vi "Multi-Record Acquisition (Fetch All records)_4xI16_7965R.vi"() -> ()   [LabVIEW 2012]
uses:
  <vilib>/userdefined/High Color/nirio_resource_hc.ctl
  <vilib>/FPGAPlugInAG/PXIe-7965R/niLvFpga_Open_PXIe-7965R.vi
  <vilib>/rvi/interface/common/dynamic/niFpgaDynamicAddResources.vi
  <vilib>/FPGAPlugInAG/Dynamic/niLvFpga_Download_Dynamic.vi
  <vilib>/FPGAPlugInAG/Dynamic/niLvFpga_Run_Dynamic.vi
  <vilib>/Utility/error.llb/Error Cluster From Error Code.vi
  <vilib>/rvi/errors/niLvFpgaAdjustHostInterfaceError.vi
  <vilib>/FPGAPlugInAG/Dynamic/niLvFpga_Close_Dynamic.vi
  <vilib>/rvi/interface/nirviOpenFPGA/nirviOpenFPGA.xnode
  <userlib>/Fast OCT/Debug/Version 1/FPGA Bitfiles/Current/Acquire 2 channel data with DRAM (Multi-Record)_latest.lvbitx
  <vilib>/rvi/interface/nirviMethod/nirviMethod.xnode
  <vilib>/rvi/interface/nirviReadWriteControl/nirviReadWriteControl.xnode
  <vilib>/rvi/interface/nirviCloseFPGA/nirviCloseFPGA.xnode
  <userlib>/FlexRIO Host Library/FlexRIO Host Library (User).lvlib
  <vilib>/rvi/interface/Simulation/niFpgaSimulationCallBeginRW.vi
  NiFpgaLv.dll
panel:
  out "Host FIFO Timed Out?":bool
  out "Buffer Timed Out?":bool
  out "Records Done":u32=500
  out "Elements Remaining":u32
  out "Iterations":i32=4
  in  "Display Raw Data?":bool=TRUE
  out "Channel Data":dbl[][](graph)
  out "Processing Time":u32=2246 format="%.0f ms"
  out "B-Scan Data":dbl[][](graph)
  in  "Device Name":T1="RIO0"
  in  "Stop":bool
  in  "Trigger Type":T2(ring)=enum."External Digital Trigger"
  in  "Record Count":u32=500
  in  "Pre Trigx4":u32=2
  in  "Post  x4":u32=1625
  out "error out":errorcluster
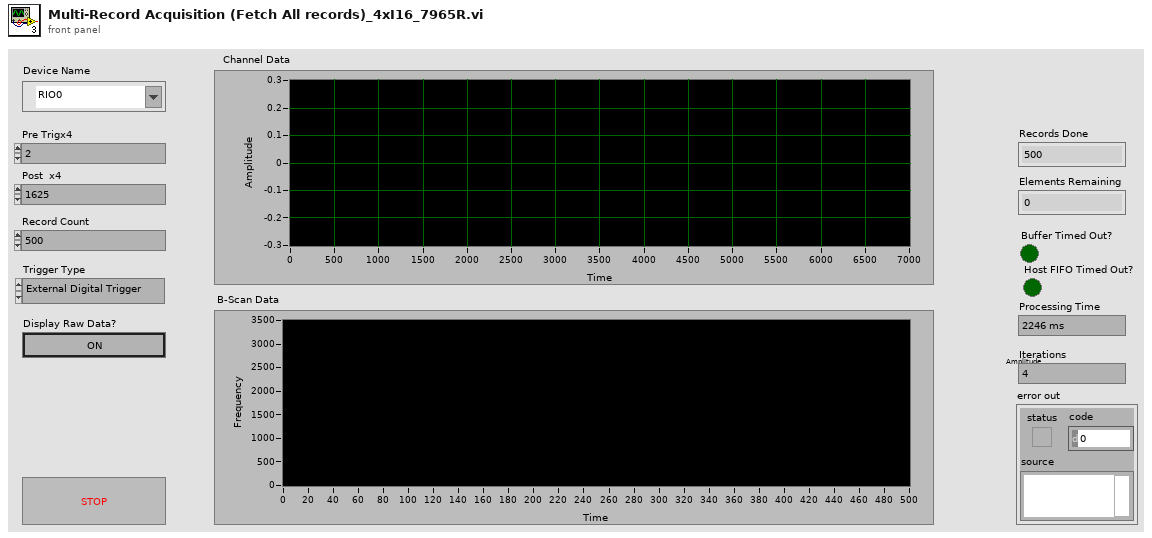
[diagram p1: front panel]
types:
  T1 = typedef "nirio_resource_hc.ctl" = tag
  T2 = enum8{"Immediate Trigger", "Software Trigger", "External Digital Trigger", "Analog Trigger"}
  T3 = cluster{"Load Record Parameters?":bool, "Pre Trigger Samples":u32, "Post Trigger Samples":u32, "Trigger Hold Off":u32, "Record Count":u32}
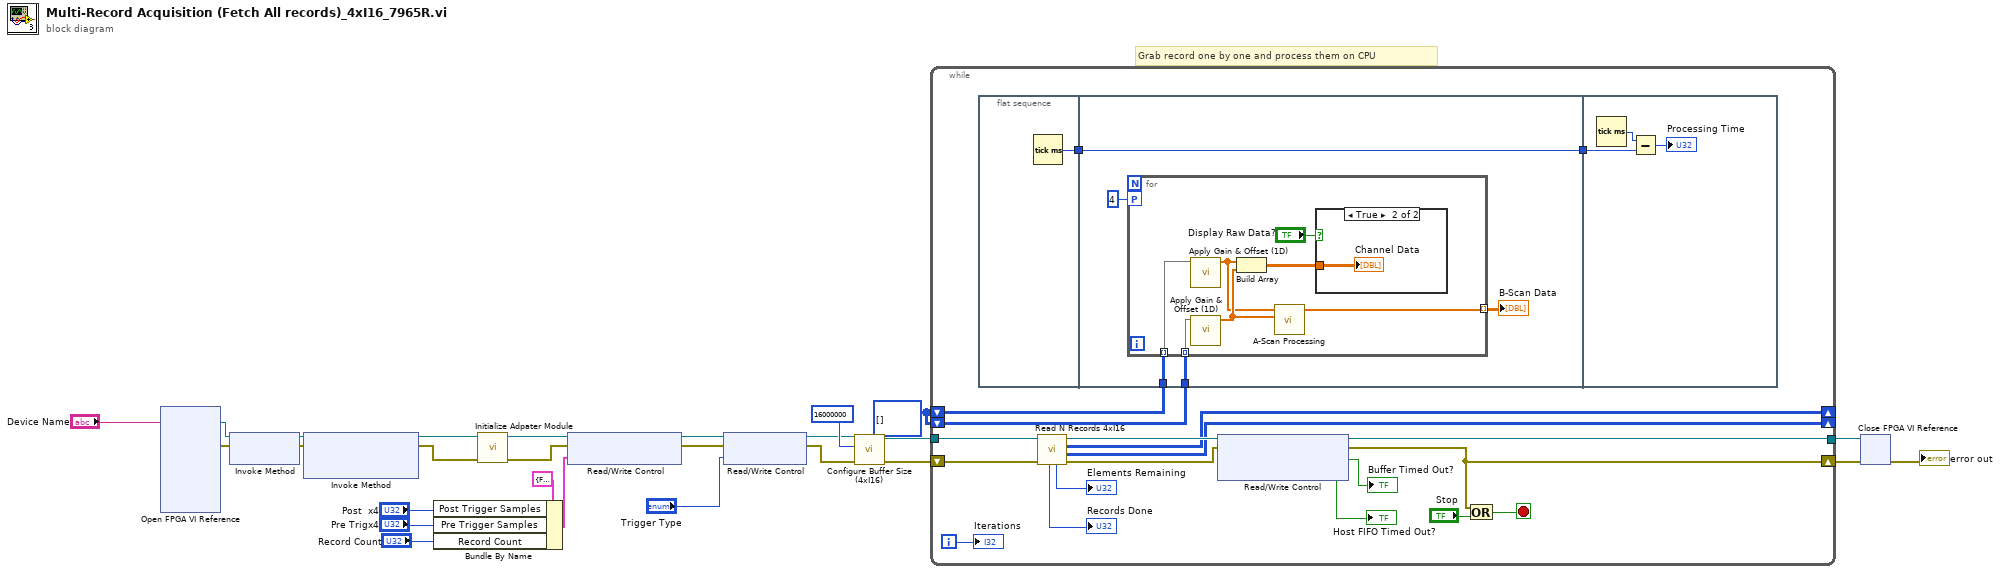
[diagram p0: block diagram]
diagram:
  w1 = i16[][] [] ("Channel 0 Records")
  # "Grab record one by one and process them on CPU"
  n1 = xnode "Open FPGA VI Reference"("resource name"="Device Name") -> ("FPGA VI Reference Out"=w8:refnum<k20>, "error out"=w9:errorcluster)  [unwired: 1 in]
  n2 = xnode "Invoke Method"("FPGA VI Reference In"=w8, "error in"=w9) -> ("FPGA VI Reference Out"=w11:refnum<k20>, "error out"=w10:errorcluster)
  n3 = xnode "Invoke Method"("FPGA VI Reference In"=w11, "error in"=w10) -> ("FPGA VI Reference Out"=w22:refnum<k20>, "error out"=w21:errorcluster)  [unwired: 1 in]
  n4 = Bundle By Name(cluster=T3 {"Load Record Parameters?"=FALSE, "Pre Trigger Samples"=0, "Post Trigger Samples"=0, "Trigger Hold Off"=0, "Record Count"=0} ("Record Parameters"), "Post Trigger Samples"="Post  x4", "Pre Trigger Samples"="Pre Trigx4", "Record Count"="Record Count") -> (w6:T3)
  n5 = call <userlib>:"Initialize Adpater Module.vi"("error in"=w21, "FPGA VI Reference In"=w22) -> ("error out"=w24:errorcluster, "FPGA VI Reference Out"=w25:refnum<k20>)  [unwired: 7 in, 1 out]
  n6 = xnode "Read/Write Control"("FPGA VI Reference In"=w25, "error in"=w24, "Record Parameters"=w6) -> ("FPGA VI Reference Out"=w19:refnum<k20>, "error out"=w18:errorcluster)
  n7 = xnode "Read/Write Control"("FPGA VI Reference In"=w19, "error in"=w18, "Trigger Type"="Trigger Type") -> ("FPGA VI Reference Out"=w14:refnum<k20>, "error out"=w15:errorcluster)
  n8 = call <userlib>:"Configure Buffer Size (4xI16).vi"("error in"=w15, "Buffer Size"=u32 16000000, "FPGA VI Reference In"=w14) -> ("error out"=w4:errorcluster, "FPGA VI Reference Out"=w5:refnum<k20>)  [unwired: 7 in]
  n9 = while {
    tunnel: w5 -> [w45]
    tunnel: [w33] -> w2
    shift-right: [w34] -> w3
    shift-left: w4 -> [w44]
    shift-right: [w30] -> _
    shift-left: w1 -> [w27]
    shift-right: [w29] -> _
    shift-left: w1 -> [w28]
    i -> [w39]
    stop <- w42 stop-if-true
    n10 = flat-sequence {
      tunnel: [w46] -> w41
      tunnel: w41 -> [w50]
      tunnel: [w50] -> w40
      tunnel: w28 -> [w49]
      tunnel: w27 -> [w48]
      tunnel: w40 -> [w61]
      frame #0 {
        n11 = Tick Count (ms)() -> (millisecond timer value=w46:u32)
      }
      frame #1 {
        n12 = for {
          tunnel: [w58] -> w51 mode=indexing
          tunnel: w49 -> [w53] mode=indexing
          tunnel: w48 -> [w52] mode=indexing
          workers-P: 4 -> [_]
          n13 = call <userlib>:"Apply Gain & Offset (1D).vi"("Raw Data"=w53) -> ("Scaled Data"=w55:dbl[])  [unwired: 10 in]
          n14 = call <userlib>:"Apply Gain & Offset (1D).vi"("Raw Data"=w52) -> ("Scaled Data"=w57:dbl[])  [unwired: 10 in]
          n15 = Build Array(w55, w57) -> (w56:dbl[][])
          n16 = call <userlib>:"A-Scan Processing.vi"("K-Clock"=w57, "OCT Signal"=w55) -> ("A-Scan"=w58:dbl[])  [unwired: 9 in]
          n17 = case shown="True" "Display Raw Data?" {
            tunnel: w56 -> [_ w59]
            frame False {
            }
            frame True {
              "Channel Data" <- w59
            }
          }
        }
        "B-Scan Data" <- w51
      }
      frame #2 {
        n18 = Tick Count (ms)() -> (millisecond timer value=w62:u32)
        n19 = Subtract(x=w62, y=w61) -> (x-y=→"Processing Time":u32)
      }
    }
    n20 = call <userlib>:"Read N Records 4xI16.vi"("error in"=w44, "FPGA VI Reference In"=w45) -> ("error out"=w35:errorcluster, "Channel 1 Records"=w30:i16[][], "Channel 0 Records"=w29:i16[][], "FPGA VI Reference Out"=w36:refnum<k20>, "Elements Remaining"=→"Elements Remaining":u32, "Records Done"=→"Records Done":u32)  [unwired: 4 in]
    n21 = xnode "Read/Write Control"("FPGA VI Reference In"=w36, "error in"=w35) -> ("FPGA VI Reference Out"=w33:refnum<k20>, "error out"=w34:errorcluster, "Buffer Timed Out?"=→"Buffer Timed Out?":bool, "Host FIFO Timed Out?"=→"Host FIFO Timed Out?":bool)
    n22 = Compound Arithmetic op=OR(w34, "Stop") -> (w42:bool)
    "Iterations" <- w39
  }
  n23 = xnode "Close FPGA VI Reference"("FPGA VI Reference In"=w2, "error in"=w3) -> ("error out"=→"error out":errorcluster)
